vi "UHR-Fleezers Control (host) - 12.7d.vi"() -> ()   [LabVIEW 2012] (continued)
                                n2052 = case shown="True" w2961 {
                                tunnel: w2978 -> [_ w2993]
                                tunnel: w2977 -> [_ w2992]
                                tunnel: w2976 -> [_ w2982]
                                tunnel: w2975 -> [_ w2984]
                                frame False {
                                }
                                frame True {
                                n2053 = local read "Time (s)"() -> (w2983:dbl)
                                n2054 = case shown="\"Yank\"" w2992 {
                                tunnel: w2993 -> [_ w2996]
                                tunnel: w2984 -> [_ w2994]
                                frame "Image", Default {
                                }
                                frame "Yank" {
                                n2055 = flat-sequence {
                                tunnel: [w3002] -> w2997
                                tunnel: w2996 -> [w3002]
                                tunnel: [w2998] -> w2995
                                tunnel: w2994 -> [w2998]
                                tunnel: w2997 -> [w3005]
                                tunnel: w2995 -> [w3003]
                                frame #0 {
                                n2056 = local read "Yank Delay (s)"() -> (w3001:dbl)
                                n2057 = Multiply(x=w3001, y=1000.0) -> (x*y=w2999:dbl)
                                n2058 = Wait (ms)(milliseconds to wait=w2999) -> ()  [unwired: 1 out]
                                }
                                frame #1 {
                                n2059 = local read "Yank to which?"() -> (w3004:bool)
                                n2060 = case shown="False" w3004 {
                                tunnel: w3005 -> [_ w3032]
                                tunnel: w3003 -> [w3006 _]
                                frame False {
                                n2061 = flat-sequence {
                                tunnel: w3006 -> [w3007]
                                frame #0 {
                                n2062 = property on="Trap Pos FB SP" class="DigNum (strict)"("Val(Sgnl)"=w3007) -> ()  [unwired: 2 in, 2 out]
                                }
                                frame #1 {
                                n2063 = Wait (ms)(milliseconds to wait=u32 700) -> ()  [unwired: 1 out]
                                }
                                frame #2 {
                                n2064 = local read "Action (%)"() -> (w3012:dbl)
                                n2065 = Absolute Value(x=w3012) -> (abs(x)=w3011:dbl)
                                n2066 = Greater?(x=w3011, y=70.0) -> (0:w3009:bool)
                                n2067 = property on="Remove Action Offset" class="Bool (strict)"("Val(Sgnl)"=w3009) -> ()  [unwired: 2 in, 2 out]
                                }
                                frame #3 {
                                n2068 = for {
                                N: 4 -> [_]
                                n2069 = flat-sequence {
                                frame #0 {
                                n2070 = Wait (ms)(milliseconds to wait=u32 500) -> ()  [unwired: 1 out]
                                }
                                frame #1 {
                                n2071 = local read "Action (%)"() -> (w3018:dbl)
                                n2072 = Absolute Value(x=w3018) -> (abs(x)=w3017:dbl)
                                n2073 = Greater?(x=w3017, y=70.0) -> (0:w3015:bool)
                                n2074 = property on="Remove Action Offset" class="Bool (strict)"("Val(Sgnl)"=w3015) -> ()  [unwired: 2 in, 2 out]
                                }
                                }
                                }
                                }
                                frame #4 {
                                n2075 = local read "Shift confocal"() -> (w3023:bool)
                                n2076 = local read "Mean"() -> (w3025:dbl)
                                n2077 = Greater?(x=w3025, y=11.0) -> (0:w3022:bool)
                                n2078 = Not(x=w3022) -> (.not. x?=w3021:bool)
                                n2079 = And(x=w3022, y=w3023) -> (x .and. y?=w3020:bool)
                                n2080 = And(x=w3021, y=w3023) -> (x .and. y?=w3019:bool)
                                n2081 = case shown="True" w3020 {
                                frame False {
                                }
                                frame True {
                                n2082 = local read "Confocal Y 2 (V)"() -> (w3029:dbl)
                                n2083 = local read "Confocal X 2 (V)"() -> (w3028:dbl)
                                n2084 = property on="AO2" class="Slide (strict)"("Val(Sgnl)"=w3028) -> ()  [unwired: 2 in, 2 out]
                                n2085 = property on="AO1" class="Slide (strict)"("Val(Sgnl)"=w3029) -> ()  [unwired: 2 in, 2 out]
                                }
                                }
                                n2086 = case shown="True" w3019 {
                                frame False {
                                }
                                frame True {
                                n2087 = local read "Confocal X 1 (V)"() -> (w3026:dbl)
                                n2088 = local read "Confocal Y 1 (V)"() -> (w3027:dbl)
                                n2089 = property on="AO1" class="Slide (strict)"("Val(Sgnl)"=w3027) -> ()  [unwired: 2 in, 2 out]
                                n2090 = property on="AO2" class="Slide (strict)"("Val(Sgnl)"=w3026) -> ()  [unwired: 2 in, 2 out]
                                }
                                }
                                }
                                frame #5 {
                                n2091 = Wait (ms)(milliseconds to wait=u32 1500) -> ()  [unwired: 1 out]
                                }
                                frame #6 {
                                n2092 = property on="Rem fb disp offset" class="Bool (strict)"("Val(Sgnl)"=TRUE ("Value (Signaling)")) -> ()  [unwired: 2 in, 2 out]
                                }
                                }
                                }
                                frame True {
                                n2093 = flat-sequence {
                                tunnel: w3032 -> [w3033]
                                frame #0 {
                                n2094 = property on="Trap Delta (MHz)" class="DigNum (strict)"("Val(Sgnl)"=w3033) -> ()  [unwired: 2 in, 2 out]
                                }
                                frame #1 {
                                n2095 = Wait (ms)(milliseconds to wait=u32 500) -> ()  [unwired: 1 out]
                                }
                                frame #2 {
                                n2096 = local read "Shift confocal"() -> (w3039:bool)
                                n2097 = local read "Mean"() -> (w3041:dbl)
                                n2098 = Greater?(x=w3041, y=11.0) -> (0:w3038:bool)
                                n2099 = Not(x=w3038) -> (.not. x?=w3037:bool)
                                n2100 = And(x=w3038, y=w3039) -> (x .and. y?=w3036:bool)
                                n2101 = And(x=w3037, y=w3039) -> (x .and. y?=w3035:bool)
                                n2102 = case shown="True" w3036 {
                                frame False {
                                }
                                frame True {
                                n2103 = local read "Confocal Y 2 (V)"() -> (w3045:dbl)
                                n2104 = local read "Confocal X 2 (V)"() -> (w3044:dbl)
                                n2105 = property on="AO2" class="Slide (strict)"("Val(Sgnl)"=w3044) -> ()  [unwired: 2 in, 2 out]
                                n2106 = property on="AO1" class="Slide (strict)"("Val(Sgnl)"=w3045) -> ()  [unwired: 2 in, 2 out]
                                }
                                }
                                n2107 = case shown="True" w3035 {
                                frame False {
                                }
                                frame True {
                                n2108 = local read "Confocal Y 1 (V)"() -> (w3043:dbl)
                                n2109 = local read "Confocal X 1 (V)"() -> (w3042:dbl)
                                n2110 = property on="AO2" class="Slide (strict)"("Val(Sgnl)"=w3042) -> ()  [unwired: 2 in, 2 out]
                                n2111 = property on="AO1" class="Slide (strict)"("Val(Sgnl)"=w3043) -> ()  [unwired: 2 in, 2 out]
                                }
                                }
                                }
                                }
                                }
                                }
                                }
                                }
                                }
                                }
                                n2112 = local read "Messages"() -> (w2991:string)
                                n2113 = Subtract(x=w2983, y=w2982) -> (x-y=w2989:dbl)
                                "Duration (s)" <- w2989
                                n2114 = Number To Decimal String(number=w2989, width (-)=i16 0) -> (decimal integer string=w2987:string)
                                n2115 = Concatenate Strings(w2987, " s fluorescence event." ("string")) -> (w2985:string)
                                n2116 = call "Update messages.vi"("Message to add"=w2985, "Old message string"=w2991) -> ("New message string"=w2990:string)
                                n2117 = local write "Reset Force"(FALSE ("Reset Force")) -> ()
                                n2118 = local write "Waiting"(TRUE ("Waiting")) -> ()
                                n2119 = local write "Messages"(w2990) -> ()
                                n2120 = local write "Fl. High"(FALSE ("Fl. High")) -> ()
                                n2121 = call <vilib>:"Beep.vi"() -> ()  [unwired: 3 in, 9 out]
                                }
                                }
                                n2122 = node-c288() -> ()  [unwired: 2 out]
                              }
                              n2123 = node-c288(w2959) -> ()  [unwired: 1 out]
                            }
                          }
                        }
                      }
                      n2124 = local read "Trap Delta (MHz)"() -> (w2874:dbl)
                      n2125 = local read "Trap Pos FB SP"() -> (w2869:fxp<+/-,16,1>)
                    }
                  }
                }
                frame #1 {
                  n2126 = local read "Stop All"() -> (w3055:bool)
                  n2127 = local read "Fl. Triggered..."() -> (w3053:bool)
                  n2128 = Not(x=w3053) -> (.not. x?=w3054:bool)
                  n2129 = Or(x=w3054, y=w3055) -> (x .or. y?=w3052:bool)
                }
              }
              n2130 = case shown="True" w2646 {
                frame False {
                }
                frame True {
                  n2131 = local read "Confocal Y 1 (V)"() -> (w2656:dbl)
                  n2132 = local read "Confocal X 1 (V)"() -> (w2655:dbl)
                  n2133 = property on="AO2" class="Slide (strict)"("Val(Sgnl)"=w2655) -> ()  [unwired: 2 in, 2 out]
                  n2134 = property on="AO1" class="Slide (strict)"("Val(Sgnl)"=w2656) -> ()  [unwired: 2 in, 2 out]
                }
              }
              n2135 = case shown="True" w2646 {
                frame False {
                }
                frame True {
                  w2654 = FALSE ("Fl. High")
                  n2136 = local write "Waiting"(w2654) -> ()
                  n2137 = local write "Fl. High"(w2654) -> ()
                }
              }
              n2138 = node-c288() -> ()  [unwired: 2 out]
            }
            n2139 = node-c288(w2644) -> ()  [unwired: 1 out]
          }
        }
      }
      event "Stop All": Value Change {
        n2140 = event-data() -> ()  [unwired: 7 out]
        n2141 = local read "Stop All"() -> (w3060:bool)
      }
    }
    n2142 = node-c288() -> ()  [unwired: 2 out]
  }
  n2143 = timed-loop "Mouse control: trap position (AOM deflection), set confocal spot from image" {
    tunnel: [w3062] -> w74
    timing: w68 -> [_]
    timing-out: [_] -> w67
    tunnel: w5 -> [w3061]
    stop <- w3062 stop-if-true
    n2144 = node-c288() -> ()  [unwired: 2 out]
    n2145 = event shown="[0] \"Pane\": Mouse Down" {
      selector: _ -> [_ _]
      dyn-events: _ -> [_ _]
      timeout: _ -> [_ _]
      tunnel: w3061 -> [w3065 _]
      event Mouse Down {
        n2146 = event-data() -> ("Time"=w3067:u32, "Coords"=w3066:T7, "Button"=w3068:u16)  [unwired: 6 out]
        n2147 = case shown="3" w3068 {
          tunnel: w3067 -> [_ _ w3174]
          tunnel: w3066 -> [_ w3105 w3172]
          tunnel: w3065 -> [_ _ w3168]
          frame 0, Default {
          }
          frame 1 {
            n2148 = property on="APD 2" class="ImageControl"() -> ("Displayed Image Position"=w3075:cluster{"Left":i32, "Top":i32})  [unwired: 2 in, 2 out]
            n2149 = property on="APD 1" class="ImageControl"() -> ("Displayed Image Position"=w3104:cluster{"Left":i32, "Top":i32})  [unwired: 2 in, 2 out]
            n2150 = property on="Detection Laser X" class="ImageControl"() -> ("Displayed Image Position"=w3101:cluster{"Left":i32, "Top":i32})  [unwired: 2 in, 2 out]
            n2151 = property on="Detection Laser Y" class="ImageControl"() -> ("Displayed Image Position"=w3100:cluster{"Left":i32, "Top":i32})  [unwired: 2 in, 2 out]
            n2152 = property on="APD 2" class="ImageControl"() -> ("Displayed Image Size"=w3074:cluster{"Width":u32, "Height":u32})  [unwired: 2 in, 2 out]
            n2153 = property on="APD 1" class="ImageControl"() -> ("Displayed Image Size"=w3102:cluster{"Width":u32, "Height":u32})  [unwired: 2 in, 2 out]
            n2154 = property on="Detection Laser X" class="ImageControl"() -> ("Displayed Image Size"=w3103:cluster{"Width":u32, "Height":u32})  [unwired: 2 in, 2 out]
            n2155 = property on="Detection Laser Y" class="ImageControl"() -> ("Displayed Image Size"=w3099:cluster{"Width":u32, "Height":u32})  [unwired: 2 in, 2 out]
            n2156 = Unbundle By Name(w3074) -> ("Width"=w3071:u32, "Height"=w3070:u32)
            n2157 = Unbundle By Name(w3075) -> ("Left"=w3073:i32, "Top"=w3072:i32)
            n2158 = Unbundle By Name(w3102) -> ("Width"=w3096:u32, "Height"=w3095:u32)
            n2159 = Unbundle By Name(w3103) -> ("Width"=w3092:u32, "Height"=w3091:u32)
            n2160 = Unbundle By Name(w3099) -> ("Width"=w3088:u32, "Height"=w3087:u32)
            n2161 = Unbundle By Name(w3104) -> ("Left"=w3098:i32, "Top"=w3097:i32)
            n2162 = Unbundle By Name(w3101) -> ("Left"=w3094:i32, "Top"=w3093:i32)
            n2163 = Unbundle By Name(w3100) -> ("Left"=w3090:i32, "Top"=w3089:i32)
            n2164 = Bundle("Left"=w3073, "Top"=w3072, "Width"=w3071, "Height"=w3070) -> (w3069:T33)  [unwired: 1 in]
            n2165 = Bundle("Left"=w3098, "Top"=w3097, "Width"=w3096, "Height"=w3095) -> (w3086:T33)  [unwired: 1 in]
            n2166 = Bundle("Left"=w3094, "Top"=w3093, "Width"=w3092, "Height"=w3091) -> (w3085:T33)  [unwired: 1 in]
            n2167 = Bundle("Left"=w3090, "Top"=w3089, "Width"=w3088, "Height"=w3087) -> (w3084:T33)  [unwired: 1 in]
            n2168 = Build Cluster Array(w3069, w3086, w3085, w3084) -> (w3083:T34)
            n2169 = for {
              tunnel: w3105 -> [w3116]
              tunnel: w3083 -> [w3117] mode=indexing
              shift-right: [w3114] -> w3081
              shift-left: TRUE -> [w3115]
              shift-right: [w3113] -> w3079
              shift-left: _ -> [w3109]
              shift-right: [w3112] -> w3078
              shift-left: _ -> [w3108]
              shift-right: [w3111] -> w3077
              shift-left: _ -> [w3107]
              shift-right: [w3110] -> w3076
              shift-left: _ -> [w3106]
              n2170 = case shown="True" w3115 {
                selector: w3115 -> [w3122 _]
                tunnel: w3117 -> [_ w3131]
                tunnel: w3116 -> [_ w3129]
                tunnel: [w3122 w3127] -> w3114
                tunnel: [w3121 w3126] -> w3113
                tunnel: [w3120 w3125] -> w3112
                tunnel: [w3119 w3124] -> w3111
                tunnel: [w3118 w3123] -> w3110
                tunnel: w3109 -> [w3121 _]
                tunnel: w3108 -> [w3120 _]
                tunnel: w3107 -> [w3119 _]
                tunnel: w3106 -> [w3118 _]
                frame False {
                }
                frame True {
                  n2171 = Unbundle(w3131) -> (w3130:T33)
                  n2172 = call "isclickinwindow.vi"("Image Param"=w3130, "Point32"=w3129) -> ("4 Y"=w3123:i32, "3 Height"=w3124:i32, "2 X"=w3125:i32, "1 Width"=w3126:i32, "In image?"=w3128:bool)  [unwired: 1 in]
                  n2173 = Not(x=w3128) -> (.not. x?=w3127:bool)
                }
              }
            }
            n2174 = Not(x=w3081) -> (.not. x?=w3080:bool)
            n2175 = case shown="True" w3080 {
              tunnel: w3078 -> [_ w3145]
              tunnel: w3076 -> [_ w3144]
              tunnel: w3079 -> [_ w3143]
              tunnel: w3077 -> [_ w3142]
              frame False {
              }
              frame True {
                w3132 = FALSE ("Get Point")
                n2176 = local read "Scan lines (y)"() -> (w3147:u64)
                n2177 = disable-structure shown="Disabled" {
                  frame Disabled {
                  }
                  frame Enabled {
                  }
                }
                n2178 = local read "Actual MCL Inc (V)"() -> (w3141:dbl)
                n2179 = local read "Scan steps (MCL)"() -> (w3146:u64)
                n2180 = Divide "Y Pix/step"(x=w3142, y=w3147) -> (x/y=w3154:dbl)
                n2181 = Divide "Y V/pix"(x=w3141, y=w3154) -> (x/y=w3153:dbl)
                n2182 = Divide "Y half step offset"(x=w3141, y=2.0) -> (x/y=w3155:dbl)
                n2183 = Divide "X pix/step"(x=w3143, y=w3146) -> (x/y=w3152:dbl)
                n2184 = Negate(x=w3155) -> (-x=w3156:dbl)
                n2185 = local read "Initial Y"() -> (w3162:dbl)
                n2186 = Multiply(x=w3144, y=w3153) -> (x*y=w3163:dbl)
                n2187 = Divide "X half step offset"(x=w3141, y=2.0) -> (x/y=w3149:dbl)
                n2188 = Divide "X V/pix"(x=w3141, y=w3152) -> (x/y=w3151:dbl)
                n2189 = Multiply(x=w3141, y=w3146) -> (x*y=w3158:dbl)
                n2190 = Compound Arithmetic op=ADD(w3156, w3163, w3162) -> (w3133:dbl)
                "Pointer Y (V)" <- w3133
                n2191 = Multiply(x=w3151, y=w3145) -> (x*y=w3160:dbl)
                n2192 = Negate(x=w3149) -> (-x=w3148:dbl)
                n2193 = local read "Initial X"() -> (w3161:dbl)
                n2194 = Negate(x=w3160) -> (-x=w3159:dbl)
                n2195 = Compound Arithmetic op=ADD(w3148, w3158, w3161, w3159) -> (w3134:dbl)
                "Pointer X (V)" <- w3134
                n2196 = case shown="True" "Set High F Confocal Spot (X-Y)" {
                  tunnel: w3134 -> [_ w3164]
                  tunnel: w3133 -> [_ w3165]
                  frame False {
                  }
                  frame True {
                    "Confocal Y 2 (V)" <- w3165
                    "Confocal X 2 (V)" <- w3164
                  }
                }
                n2197 = Or(x="Set X Only", y="Set Confocal Spot (X-Y)") -> (x .or. y?=w3137:bool)
                n2198 = Or(x="Set Confocal Spot (X-Y)", y="Set Y Only") -> (x .or. y?=w3136:bool)
                n2199 = case shown="True" w3137 {
                  tunnel: w3134 -> [_ w3166]
                  frame False {
                  }
                  frame True {
                    n2200 = property on="AO2" class="Slide (strict)"("Val(Sgnl)"=w3166) -> ()  [unwired: 2 in, 2 out]
                    "Confocal X 1 (V)" <- w3166
                  }
                }
                n2201 = case shown="True" w3136 {
                  tunnel: w3133 -> [_ w3167]
                  frame False {
                  }
                  frame True {
                    n2202 = property on="AO1" class="Slide (strict)"("Val(Sgnl)"=w3167) -> ()  [unwired: 2 in, 2 out]
                    "Confocal Y 1 (V)" <- w3167
                  }
                }
                n2203 = local write "Set High F Confocal Spot (X-Y)"(w3132) -> ()
                n2204 = local write "Set Confocal Spot (X-Y)"(w3132) -> ()
                n2205 = local write "Set X Only"(w3132) -> ()
                n2206 = local write "Set Y Only"(w3132) -> ()
              }
            }
          }
          frame 3 {
            n2207 = local read "BD 2 Frequency 1 (MHz)"() -> (w3169:dbl)
            n2208 = local read "BD 1 Frequency 1 (MHz)"() -> (w3170:dbl)
            n2209 = local write "Manipulating Trap"(TRUE ("Manipulating Trap")) -> ()
            n2210 = local write "Coords"(T7 {"Horizontal"=0, "Vertical"=0} ("Coords")) -> ()
            n2211 = while {
              tunnel: w3174 -> [w3179]
              tunnel: w3172 -> [w3178]
              tunnel: w3170 -> [w3177]
              tunnel: w3169 -> [w3176]
              tunnel: w3168 -> [w3175]
              stop <- w3180 stop-if-true
              n2212 = event shown="[0] \"Pane\": Mouse Move" {
                selector: _ -> [_ _]
                dyn-events: _ -> [_ _]
                timeout: _ -> [_ _]
                tunnel: ["Force Manip Abort" w3244] -> w3180
                tunnel: w3179 -> [w3187 _]
                tunnel: w3178 -> [w3185 _]
                tunnel: w3177 -> [w3184 _]
                tunnel: w3176 -> [w3183 _]
                tunnel: w3175 -> [w3181 _]
                event Mouse Move {
                  n2213 = event-data() -> ("Time"=w3188:u32, "Coords"=w3189:T7)  [unwired: 3 out]
                  n2214 = Less?(x=w3188, y=w3187) -> (x < y?=w3186:bool)
                  n2215 = case "Makes sure old motion events prior to mouse click aren't used" shown="False" w3186 {
                    tunnel: w3189 -> [w3231 _]
                    tunnel: w3185 -> [w3232 _]
                    tunnel: w3184 -> [w3206 _]
                    tunnel: w3183 -> [w3205 _]
                    tunnel: w3181 -> [w3190 _]
                    frame False {
                      n2216 = Subtract(x=w3231, y=w3232) -> (x-y=w3230:T7)
                      "Coords" <- w3230
                      n2217 = local read "Y RF Frequency Limits (MHz)"() -> (w3191:T16)
                      n2218 = To Double Precision Float(number=w3230) -> (double precision float=w3229:cluster{"Horizontal":dbl, "Vertical":dbl})
                      n2219 = Multiply(x=cluster{"Horizontal":dbl, "Vertical":dbl} {"Horizontal"=-1.0, "Vertical"=1.0}, y="Manipulation Scaling") -> (x*y=w3225:cluster{"Horizontal":dbl, "Vertical":dbl})
                      n2220 = local read "X RF Frequency Limits (MHz)"() -> (w3192:T16)
                      n2221 = Multiply(x=w3229, y=w3225) -> (x*y=w3227:cluster{"Horizontal":dbl, "Vertical":dbl})
                      n2222 = Unbundle By Name(w3227) -> ("Horizontal"=w3222:dbl, "Vertical"=w3226:dbl)
                      n2223 = Unbundle By Name(w3191) -> ("Maximum"=w3194:dbl, "Minimum"=w3193:dbl)
                      n2224 = Boolean To (0,1)(Boolean="Manip. X?") -> (0, 1=w3220:i16)
                      n2225 = Boolean To (0,1)(Boolean="Manip. Y?") -> (0, 1=w3217:i16)
                      n2226 = local read "BD 1 Frequency 2 (MHz)"() -> (w3208:dbl)
                      n2227 = Multiply(x=w3226, y=w3217) -> (x*y=w3219:dbl)
                      n2228 = Multiply(x=w3220, y=w3222) -> (x*y=w3223:dbl)
                      n2229 = local read "BD 2 Frequency 2 (MHz)"() -> (w3207:dbl)
                      n2230 = Unbundle By Name(w3192) -> ("Maximum"=w3196:dbl, "Minimum"=w3195:dbl)
                      n2231 = Add(x=w3205, y=w3219) -> (x+y=w3198:dbl)
                      n2232 = Add(x=w3206, y=w3223) -> (x+y=w3200:dbl)
                      n2233 = In Range and Coerce(upper limit=w3196, x=w3200, lower limit=w3195) -> (coerced(x)=w3199:dbl)  [unwired: 1 out]
                      n2234 = In Range and Coerce(upper limit=w3194, x=w3198, lower limit=w3193) -> (coerced(x)=w3197:dbl)  [unwired: 1 out]
                      n2235 = Subtract(x=w3199, y=w3208) -> (x-y=w3216:dbl)
                      n2236 = Subtract(x=w3197, y=w3207) -> (x-y=w3215:dbl)
                      n2237 = Square(x=w3216) -> (x^2=w3214:dbl)
                      n2238 = Square(x=w3215) -> (x^2=w3213:dbl)
                      n2239 = Add(x=w3214, y=w3213) -> (x+y=w3212:dbl)
                      n2240 = Square Root(x=w3212) -> (sqrt(x)=w3209:dbl)
                      n2241 = In Range and Coerce(upper limit="Limit Max (MHz)", x=w3209, lower limit="Limit Min (MHz)") -> (In Range?=w3202:bool)  [unwired: 1 out]
                      n2242 = Not(x="Limits Enable") -> (.not. x?=w3201:bool)
                      n2243 = Or(x=w3202, y=w3201) -> (x .or. y?=w3203:bool)
                      n2244 = case shown="True" w3203 {
                        tunnel: w3209 -> [_ w3234]
                        tunnel: w3199 -> [_ w3241]
                        tunnel: w3208 -> [_ w3240]
                        tunnel: w3197 -> [_ w3239]
                        tunnel: w3207 -> [_ w3238]
                        tunnel: w3192 -> [_ w3236]
                        tunnel: w3191 -> [_ w3235]
                        tunnel: w3190 -> [_ w3233]
                        frame False {
                        }
                        frame True {
                          n2245 = local read "BD 1 Frequency 3 (MHz)"() -> (w3242:dbl)
                          n2246 = local read "BD 2 Frequency 3 (MHz)"() -> (w3237:dbl)
                          n2247 = local write "Trap Delta (MHz)"(w3234) -> ()
                          n2248 = call "set RF board frequency - interlace.vi"("Board 2 Frequency Limits"=w3235, "Board 1 Frequency Limits"=w3236, "FPGA VI Reference In"=w3233, "Board 2 Frequency 3 (MHz)"=w3237, "Board 1 Frequency 3 (MHz)"=w3242, "Board 2 Frequency 2 (MHz)"=w3238, "Board 2 Frequency 1 (MHz)"=w3239, "Board 1 Frequency 2 (MHz)"=w3240, "Board 1 Frequency 1  (MHz)"=w3241) -> ()  [unwired: 1 in, 2 out]
                          n2249 = local write "BD 2 Frequency 1 (MHz)"(w3239) -> ()
                          n2250 = local write "BD 1 Frequency 1 (MHz)"(w3241) -> ()
                        }
                      }
                    }
                    frame True {
                    }
                  }
                }
                event Mouse Up {
                  n2251 = event-data() -> ("Button"=w3243:u16)  [unwired: 8 out]
                  n2252 = case shown="3" w3243 {
                    tunnel: [FALSE TRUE] -> w3244
                    frame 0, Default {
                    }
                    frame 3 {
                      n2253 = local read "Trap Delta (MHz)"() -> (w3246:dbl)
                      n2254 = property on="Initial delta (MHz)" class="DigNum (strict)"("Val(Sgnl)"=w3246) -> ()  [unwired: 2 in, 2 out]
                      n2255 = local write "Manipulating Trap"(FALSE ("Manipulating Trap")) -> ()
                    }
                  }
                }
              }
            }
          }
        }
      }
      event Mouse Move {
        n2256 = event-data() -> ()  [unwired: 6 out]
      }
    }
    n2257 = local read "Stop All"() -> (w3062:bool)
    n2258 = node-c288() -> ()  [unwired: 2 out]
  }
  n2259 = flat-sequence "Video" {
    tunnel: [w3258] -> w55
    tunnel: w55 -> [w3298]
    frame #0 {
      n2260 = while {
        stop <- w3250 continue-if-true
        n2261 = call "Close Video Capture.vi"() -> ("error code OUT"=w3252:i32)
        n2262 = Equal?(x=w3252, y=0) -> (x = y?=w3250:bool)
      }
      n2263 = local write "Stop All"(FALSE ("Stop All")) -> ()
    }
    frame #1 {
      n2264 = call "DMR_Init.vi"() -> ()  [unwired: 3 out]
    }
    frame #2 {
      w3253 = "DE245428202"  # MSU fleezers card #
      (unwired) "DE019116701"  # Illinois fleezers card #
      # "Setting the destination format to Mono8 makes sure that the image can be displayed in the intensity plot."
      n2265 = call "DMR_GetDevice.vi"("search string IN"=w3253) -> ("device handle OUT"=w3276:i32)  [unwired: 4 in, 2 out]
      n2266 = call "DMR_OpenDevice.vi"("device handle IN"=w3276) -> ("driver handle OUT"=w3259:i32)  [unwired: 4 out]
      n2267 = call "DMR_FindList.vi"("flags IN"=u32 0 ("flags"), "list name IN"="" ("String"), "list type IN"=T35."camera descriptions", "driver handle IN"=w3259) -> ("list handle OUT"=w3262:i32)  [unwired: 2 out]
      n2268 = call "DMR_FindList.vi"("flags IN"=u32 0 ("flags"), "list name IN"="Base", "list type IN"=T35."setting", "driver handle IN"=w3259) -> ("list handle OUT"=w3260:i32)  [unwired: 2 out]
      n2269 = call "OBJ_GetHandle.vi"("object name IN"="VideoStandard", "list handle IN"=w3262) -> ("object handle OUT"=w3256:i32)  [unwired: 3 out]
      n2270 = call "OBJ_GetHandle.vi"("object name IN"="PixelFormat", "list handle IN"=w3260) -> ("object handle OUT"=w3270:i32)  [unwired: 3 out]
      n2271 = call "OBJ_SetS.vi"("value index IN"=0, "value IN"="NTSC M", "object handle IN"=w3256) -> ()  [unwired: 2 out]
      n2272 = call "OBJ_SetS.vi"("value index IN"=0, "value IN"="Mono8" ("value"), "object handle IN"=w3270) -> ()  [unwired: 2 out]
      n2273 = call "OBJ_GetHandle.vi"("object name IN"="VideoChannel", "list handle IN"=w3260) -> ("object handle OUT"=w3266:i32)  [unwired: 3 out]
      n2274 = while {
        tunnel: [w3280] -> w3258
        tunnel: w3259 -> [w3277]
        stop <- w3278 continue-if-true
        n2275 = call "DMR_ImageRequestSingle.vi"("request control IN"=0, "driver handle IN"=w3277) -> ("error code OUT"=w3279:i32, "driver handle OUT"=w3280:i32)  [unwired: 2 out]
        n2276 = Equal To 0?(x=w3279) -> (x = 0?=w3278:bool)
      }
      n2277 = call "OBJ_SetI.vi"("value index IN"=0, "value IN"=3 ("Video channel"), "object handle IN"=w3266) -> ()  [unwired: 2 out]
    }
    frame #3 {
      w3286 = T19 0 items=["Grayscale (U8)", "Grayscale (I16)", "Grayscale (SGL)", "Complex (CSG)", "RGB (U32)", "HSL (U32)", "RGB (U64)"] ("Image Type")
      w3294 = T19 0 items=["Grayscale (U8)", "Grayscale (I16)", "Grayscale (SGL)", "Complex (CSG)", "RGB (U32)", "HSL (U32)", "RGB (U64)"] ("Image Type")
      n2278 = for "Create Greyscale map" {
        N: 256 -> [_]
        tunnel: [w3300] -> w3283 mode=indexing
        workers-P: _ -> [_]
        i -> [w3303]
        n2279 = To Unsigned Byte Integer(number=w3303) -> (unsigned 8bit integer=w3299:u8)
        n2280 = Join Numbers(hi=w3299, lo=w3299) -> ((hi.lo)=w3302:u16)
        n2281 = Join Numbers(hi=w3299, lo=w3299) -> ((hi.lo)=w3301:u16)
        n2282 = Join Numbers(hi=w3302, lo=w3301) -> ((hi.lo)=w3300:u32)
      }
      n2283 = call "IMAQ Create"("Image Name"="Scaled video", "Image Type"=w3286) -> ("New Image"=w3285:T2)  [unwired: 2 in, 2 out]
      n2284 = call "IMAQ Create"("Image Name"="Main video", "Image Type"=w3294) -> ("New Image"=w3295:T2)  [unwired: 2 in, 2 out]
      n2285 = node-c288(0 ("Processor")) -> (w3293:T23)  [unwired: 3 out]
      n2286 = Initialize Array(u32 0 ("Window Number (0...15)"), 480 ("dimension size"), 640 ("dimension size")) -> (w3288:u32[][])
      n2287 = timed-loop {
        tunnel: w3298 -> [w3320]
        tunnel: [w3319] -> w3297
        tunnel: w3295 -> [w3318]
        timing: w3293 -> [_]
        timing-out: [_] -> w3292
        tunnel: w3288 -> [w3307]
        tunnel: w3285 -> [w3305]
        tunnel: w3283 -> [w3304]
        stop <- w3306 stop-if-true
        # "This block performs the \nactual image capture."
        n2288 = node-c288() -> ()  [unwired: 2 out]
        n2289 = local read "Stop All"() -> (w3306:bool)
        n2290 = Reciprocal(x="Video Capture Rate (Hz)") -> (1/x=w3310:dbl)
        n2291 = Multiply(x=w3310, y=1000.0) -> (x*y=w3308:dbl)
        n2292 = call "DMR_ImageRequestWaitFor.vi"("queue number IN"=0, "timeout(ms) IN"=500, "driver handle IN"=w3320) -> ("error code OUT"=w3324:i32, "request number OUT"=w3321:i32, "driver handle OUT"=w3322:i32)
        n2293 = feedback #1(T36 refnum ("Avi Refnum")) -> (w3312:T36)
        n2294 = case shown="True" "New Video File" {
          tunnel: [T36 refnum ("Avi Refnum") w3341] -> w3314
          tunnel: [FALSE TRUE] -> w3315
          tunnel: w3312 -> [_ w3337]
          frame False {
          }
          frame True {
            n2295 = call "Create new save file.vi"("Ext"=".avi" ("string"), "Index In"="Video Index") -> ("Path Out"=w3333:path, "Index Out"=w3334:dbl)  [unwired: 1 in]
            "Path Out" <- w3333
            n2296 = Not Equal?(x=w3337, y=T36 refnum ("Avi Refnum")) -> (x != y?=w3338:bool)
            n2297 = Increment(x=w3334) -> (x+1=w3343:dbl)
            n2298 = case shown="True" w3338 {
              tunnel: w3337 -> [_ w3344]
              frame False {
              }
              frame True {
                n2299 = call "IMAQ AVI Close"("Avi Refnum"=w3344) -> ()  [unwired: 1 in, 10 out]
              }
            }
            n2300 = local write "Video Index"(w3343) -> ()
            n2301 = call "IMAQ AVI Create"("Frames Per Second"=u32 30, "AVI Path"=w3333) -> ("Avi Refnum"=w3341:T36)  [unwired: 5 in, 4 out]
          }
        }
        n2302 = Equal To 0?(x=w3324) -> (x = 0?=w3323:bool)
        n2303 = Select(t=w3314, s=w3315, f=w3312) -> (s? t:f=w3313:T36)
        n2304 = feedback-in #1(w3313) -> ()
        n2305 = case shown="True" w3323 {
          tunnel: w3322 -> [w3345 w3379]
          tunnel: w3321 -> [_ w3378]
          tunnel: [w3345 w3375] -> w3319
          tunnel: w3318 -> [_ w3360]
          tunnel: w3307 -> [_ w3364]
          tunnel: w3313 -> [_ w3362]
          tunnel: w3305 -> [_ w3357]
          tunnel: w3304 -> [_ w3356]
          frame False {
          }
          frame True {
            w3369 = u32 0 ("X-offset IN")
            n2306 = call "DMR_GetImageRequestBufferData.vi"("driver handle IN"=w3379, "request number IN"=w3378) -> ("width OUT"=w3368:i32, "height OUT"=w3367:i32, "driver handle OUT"=w3374:i32, "request number OUT"=w3373:i32, "bytes per pixel OUT"=w3370:i32)  [unwired: 13 out]
            n2307 = call "DMR_GetImageRequestBufferImageData.vi"("driver handle IN"=w3374, "request number IN"=w3373, "bytes per pixel IN"=w3370, "X-offset IN"=w3369, "Y-offset IN"=w3369, "height IN"=w3367, "width IN"=w3368) -> ("driver handle OUT"=w3372:u32, "request number OUT"=w3371:u32, "image OUT"=w3349:u32[][])  [unwired: 10 out]
            n2308 = Transpose 2D Array(2D array=w3349) -> (transposed array=w3355:u32[][])
            n2309 = Select(t=w3355, s="Flip Y (or X)", f=w3349) -> (s? t:f=w3354:u32[][])
            n2310 = call "DMR_ImageRequestUnlock.vi"("request number IN"=w3371, "driver handle IN"=w3372) -> ("driver handle OUT"=w3377:i32)  [unwired: 1 in, 2 out]
            n2311 = for {
              tunnel: w3354 -> [w3414] mode=indexing
              tunnel: [w3413] -> w3352 mode=indexing
              n2312 = Reverse 1D Array(array=w3414) -> (reversed array=w3413:u32[])
            }
            n2313 = call "DMR_ImageRequestSingle.vi"("request control IN"=0, "driver handle IN"=w3377) -> ("driver handle OUT"=w3375:i32)  [unwired: 3 out]
            n2314 = Transpose 2D Array(2D array=w3352) -> (transposed array=w3353:u32[][])
            n2315 = Select(t=w3353, s="Flip Y (or X)", f=w3352) -> (s? t:f=w3350:u32[][])
            n2316 = Select(t=w3350, s="Flip Image", f=w3349) -> (s? t:f=w3347:u32[][])
            n2317 = case shown="True" "Averaging" {
              tunnel: w3347 -> [w3417 w3422]
              tunnel: [w3417 w3421] -> w3361
              tunnel: w3364 -> [_ w3419]
              frame False {
              }
              frame True {
                (unwired) 1
                w3427 = 1
                n2318 = feedback #2(w3419) -> (w3418:u32[][])
                n2319 = Add(x=w3422, y=w3418) -> (x+y=w3423:u32[][])
                n2320 = Select(t=w3419, s="Reset Averaging", f=w3423) -> (s? t:f=w3425:u32[][])
                n2321 = feedback-in #2(w3425) -> ()
                n2322 = feedback #3(w3427) -> (w3420:i32)
                n2323 = Divide(x=w3423, y=w3420) -> (x/y=w3424:dbl[][])
                n2324 = Increment(x=w3420) -> (x+1=w3428:i32)
                n2325 = To Unsigned Long Integer(number=w3424) -> (unsigned 32bit integer=w3421:u32[][])
                n2326 = Select(t=w3427, s="Reset Averaging", f=w3428) -> (s? t:f=w3426:i32)
                n2327 = feedback-in #3(w3426) -> ()
              }
            }
            n2328 = case shown="True" "Zoom video window" {
              tunnel: w3361 -> [_ w3393]
              tunnel: w3357 -> [_ w3392]
              frame False {
              }
              frame True {
                n2329 = To Double Precision Float(number=w3393) -> (double precision float=w3390:dbl[][])
                n2330 = In Range and Coerce(upper limit="Intensity Upper", x=w3390, lower limit="Intensity Lower") -> (coerced(x)=w3389:dbl[][])  [unwired: 1 out]
                n2331 = Subtract(x="Intensity Upper", y="Intensity Lower") -> (x-y=w3386:dbl)
                n2332 = Subtract(x=w3389, y="Intensity Lower") -> (x-y=w3387:dbl[][])
                n2333 = Divide(x=w3387, y=w3386) -> (x/y=w3388:dbl[][])
                n2334 = Multiply(x=255.0, y=w3388) -> (x*y=w3384:dbl[][])
                n2335 = To Unsigned Byte Integer(number=w3384) -> (unsigned 8bit integer=w3391:u8[][])
                n2336 = call "IMAQ ArrayToImage"("Image Pixels (U8)"=w3391, "Image"=w3392) -> ("Image Out"=w3380:T2)  [unwired: 4 in, 5 out]
                n2337 = First Call?() -> (First Call?: T/F=w3381:bool)
                n2338 = case shown="True" w3381 {
                  tunnel: w3380 -> [w3394 w3405]
                  frame False {
                    n2339 = flat-sequence {
                      tunnel: w3394 -> [w3400]
                      frame #0 {
                        w3397 = FALSE ("Get/Set Status? (Set)")
                        w3396 = 0 ("Window Number (0...15)")
                        n2340 = call "IMAQ WindSize"("Get/Set Status? (Set)"=w3397, "Window Number"=w3396) -> ("Width & Height out"=→"Window Size":cluster{"Width":i32, "Height":i32})  [unwired: 4 in, 2 out]
                        n2341 = call "IMAQ WindMove"("Window Number (0...15)"=w3396, "Get/Set Status? (Set)"=w3397) -> ("Coordinates (screen)"=→"Window Position":cluster{"X Position":i32, "Y Position":i32})  [unwired: 3 in, 1 out]
                        n2342 = call "IMAQ WindDraw"("Resize to Image Size? (Y)"=FALSE, "Window Number (0...15)"=w3396, "Image"=w3400) -> ()  [unwired: 7 in, 2 out]
                      }
                      frame #1 {
                        n2343 = call "IMAQ WindZoom 2"("Center Point"="Center Point", "Zoom to Fit? (False)"=FALSE, "Zoom Factor"="Zoom Factor") -> ()  [unwired: 5 in, 4 out]
                      }
                    }
                  }
                  frame True {
                    n2344 = flat-sequence {
                      tunnel: w3405 -> [w3408]
                      tunnel: [w3406] -> w3404
                      tunnel: w3404 -> [w3410]
                      frame #0 {
                        w3407 = TRUE ("Resize to Image Size? (Y)")
                        w3406 = 0 ("Window Number (0...15)")
                        n2345 = call "IMAQ WindNonTearing"("Window Number"=w3406, "NonTearing? (True)"=w3407) -> ()  [unwired: 8 in, 2 out]
                        n2346 = call "IMAQ WindDraw"("Resize to Image Size? (Y)"=w3407, "Window Number (0...15)"=w3406, "Image"=w3408) -> ()  [unwired: 7 in, 2 out]
                      }
                      frame #1 {
                        n2347 = call "IMAQ WindSize"("Scrollbars? (N)"=FALSE, "Width & Height"="Initial Window Size", "Window Number"=w3410) -> ()  [unwired: 3 in, 3 out]
                        n2348 = call "IMAQ WindMove"("Window Number (0...15)"=w3410, "Coordinates (screen)"="Initial Window Position") -> ()  [unwired: 3 in, 2 out]
                      }
                    }
                  }
                }
              }
            }
            n2349 = To Unsigned Byte Integer(number=w3361) -> (unsigned 8bit integer=w3359:u8[][])
            n2350 = call "IMAQ ArrayToImage"("Image Pixels (U8)"=w3359, "Image"=w3360) -> ("Image Out"=w3358:T2)  [unwired: 4 in, 5 out]
            "Primary Video Display" <- w3358
            n2351 = case shown="True" "Save Video" {
              tunnel: w3362 -> [_ w3416]
              tunnel: w3358 -> [_ w3415]
              frame False {
              }
              frame True {
                n2352 = call "IMAQ AVI Write Frame"("Image"=w3415, "Avi Refnum"=w3416) -> ()  [unwired: 2 in, 8 out]
              }
            }
            n2353 = case shown="True" "Save Image" {
              tunnel: w3359 -> [_ w3431]
              tunnel: w3356 -> [_ w3430]
              frame False {
              }
              frame True {
                n2354 = call <vilib>:"Flatten Pixmap.vi"("colors"=w3430, "8-bit pixmap"=w3431) -> ("image data"=w3437:T37)  [unwired: 4 in, 5 out]
                n2355 = call "Create new save file.vi"("Insert"="video_frame_" ("string"), "Ext"=".bmp" ("string"), "Index In"="Image Index") -> ("Path Out"=w3433:path, "Index Out"=w3438:dbl)
                n2356 = Increment(x=w3438) -> (x+1=w3432:dbl)
                n2357 = local write "Image Index"(w3432) -> ()
                n2358 = call <vilib>:"Write BMP File.vi"("image data"=w3437, "path to BMP file"=w3433) -> ()  [unwired: 1 in, 9 out]
              }
            }
          }
        }
        n2359 = node-c288(w3308) -> ()  [unwired: 1 out]
      }
      n2360 = node-c288(w3292) -> ()  [unwired: 1 out]
      n2361 = call "DMR_CloseDevice.vi"("driver handle IN"=w3297) -> ()  [unwired: 1 in, 4 out]
    }
    frame #4 {
      n2362 = call "DMR_Close.vi"() -> ()  [unwired: 1 out]
    }
  }
  n2363 = node-c288(i64 1 ("Period"), 1 ("Processor")) -> (w73:T23)  [unwired: 2 out]
  n2364 = timed-loop "Main data acquisition loop (get data, process data for display, and save data to disk)" {
    tunnel: w11 -> [w3761]
    tunnel: w10 -> [w3760]
    tunnel: [w3789] -> w80
    tunnel: [w3784] -> w79
    timing: w73 -> [_]
    timing-out: [_] -> w72
    tunnel: w47 -> [w3615]
    stop <- "Stop All" stop-if-true
    w3532 = "Initialize"
    # "T2 sum"
    # "T1 sum"
    # "Fluorescence data into FIFO for external control vi's\n(e.g., fluorescence triggering) - Duncan Nall"
    n2365 = node-c288() -> ()  [unwired: 2 out]
    n2366 = First Call?() -> (First Call?: T/F=w3567:bool)
    n2367 = Or(x="Reset", y=w3567) -> (x .or. y?=w3568:bool)
    n2368 = local read "Flushing P1"() -> (w3487:bool)
    n2369 = case "Reset data stream (manual reset or at begining of some rastering and imaging)" shown="True" w3568 {
      tunnel: w3761 -> [w4830 w4838]
      tunnel: w3760 -> [w4829 w4837]
      tunnel: [w4830 w4832] -> w3756
      tunnel: [w4829 w4831] -> w3755
      frame False {
      }
      frame True {
        w4835 = TRUE ("AI to FIFO")
        n2370 = local write "Overflow (data lost)"(FALSE ("Overflow (data lost)")) -> ()
        n2371 = call "reset FPGA DMA.vi"("error in"=w4837, "FPGA VI Reference In"=w4838) -> ("error out"=w4833:errorcluster, "FPGA VI Reference Out"=w4834:T20)
        n2372 = xnode "Read/Write Control"("FPGA VI Reference In"=w4834, "error in"=w4833, "AI to FIFO"=w4835, "APD to FIFO"=w4835) -> ("FPGA VI Reference Out"=w4832:T20, "error out"=w4831:errorcluster)
      }
    }
    n2373 = case shown="True" w3487 {
      frame False {
      }
      frame True {
        n2374 = local read "Flush rate (uL/m) P1"() -> (w3819:dbl)
        n2375 = local read "HP1 Flush Time (s)"() -> (w3828:dbl)
        n2376 = local read "DMA Update Period (s)"() -> (w3822:dbl)
        n2377 = Divide(x=w3819, y=60.0) -> (x/y=w3820:dbl)
        n2378 = Divide(x=w3828, y=w3822) -> (x/y=w3817:dbl)
        n2379 = feedback #4(0) -> (w3826:i32)
        n2380 = Increment(x=w3826) -> (x+1=w3816:i32)
        n2381 = Greater?(x=w3816, y=w3817) -> (0:w3825:bool)
        n2382 = Compound Arithmetic op=MULTIPLY(w3822, w3816, w3820) -> (→"P1 Flush Volume (uL)":dbl)
        n2383 = Divide(x=w3816, y=w3817) -> (x/y=→"P1 Flushing Bar":dbl)
        n2384 = case shown="True" w3825 {
          tunnel: w3816 -> [w3829 _]
          tunnel: [w3829 0] -> w3824
          frame False {
          }
          frame True {
            w3830 = FALSE ("Flushing P1")
            n2385 = local write "Inject Pump 1"(w3830) -> ()
            n2386 = local write "Flushing P1"(w3830) -> ()
            n2387 = property on="Clear Volume P1" class="Bool (strict)"("Val(Sgnl)"=TRUE ("Value (Signaling)")) -> ()  [unwired: 2 in, 2 out]
          }
        }
        n2388 = feedback-in #4(w3824) -> ()
      }
    }
    n2389 = Or(x="Start AOD Scan", y="Trap Raster Scan") -> (x .or. y?=w3712:bool)
    n2390 = case "Start AOM raster scan" shown="True" w3712 {
      tunnel: w3756 -> [w4680 w4690]
      tunnel: w3755 -> [w4679 w4689]
      tunnel: [w4680 w4683] -> w3754
      tunnel: [w4679 w4682] -> w3753
      frame False {
      }
      frame True {
        n2391 = case shown="True" "Restart DMA? (AOD)" {
          tunnel: [w4728 w4730] -> w4684
          tunnel: [w4727 w4729] -> w4685
          tunnel: w4690 -> [w4728 w4732]
          tunnel: w4689 -> [w4727 w4731]
          frame False {
          }
          frame True {
            n2392 = local write "Overflow (data lost)"(FALSE ("Overflow (data lost)")) -> ()
            n2393 = call "reset FPGA DMA.vi"("error in"=w4731, "FPGA VI Reference In"=w4732) -> ("error out"=w4729:errorcluster, "FPGA VI Reference Out"=w4730:T20)
          }
        }
        n2394 = local write "Trap Raster Scan"(FALSE ("Trap Raster Scan")) -> ()
        n2395 = case shown="True" "Move MCL Also?" {
          tunnel: w4685 -> [w4693 w4722]
          tunnel: w4684 -> [w4694 w4723]
          tunnel: [w4692 w4726] -> w4683
          tunnel: [w4691 w4725] -> w4682
          frame False {
            w4695 = TRUE ("AI to FIFO")
            n2396 = xnode "Read/Write Control"("FPGA VI Reference In"=w4694, "error in"=w4693, "AI to FIFO"=w4695, "APD to FIFO"=w4695, "Start scan"=w4695) -> ("FPGA VI Reference Out"=w4692:T20, "error out"=w4691:errorcluster)
          }
          frame True {
            w4719 = FALSE ("1D or 2D Scan?")
            w4724 = TRUE ("AI to FIFO")
            # "Count for MCL loop"
            # "N total cycles"
            # "N steps"
            # "V_int"
            n2397 = local read "Scan Range (nm)"() -> (w4701:dbl)
            n2398 = local read "Number of F/B Scans (AOD)"() -> (w4718:u16)
            n2399 = Sign(1:w4701) -> (0:w4700:dbl)
            n2400 = Compound Arithmetic op=MULTIPLY(w4701, "MCL Step Position Ratio", "MCL/AOM Scale Tweak") -> (w4705:dbl)
            n2401 = Negate(x=w4700) -> (-x=w4697:dbl)
            n2402 = Multiply(x=w4697, y="MCL Step Increment (V_int)") -> (x*y=w4699:dbl)
            n2403 = Divide(x=w4705, y="MCL X Cal (nm/V)") -> (x/y=w4711:dbl)
            n2404 = Multiply(x=32767.0 ("y"), y=w4711) -> (x*y=w4717:dbl)
            n2405 = local read "Total Counts (ticks)"() -> (w4702:u16)
            n2406 = local read "Cycles/step (AOD)"() -> (w4713:u64)
            n2407 = local read "Scan steps (AOD)"() -> (w4714:u64)
            n2408 = Divide(x=w4717, y=10.0) -> (x/y=w4710:dbl)
            n2409 = Divide(x=w4710, y="MCL Step Increment (V_int)") -> (x/y=w4708:dbl)
            n2410 = Absolute Value(x=w4708) -> (abs(x)=w4696:dbl)
            n2411 = Compound Arithmetic op=MULTIPLY(w4714, w4713, w4702) -> (w4709:u64)
            n2412 = local write "wait to reset values"(w4724) -> ()
            n2413 = local write "MCL Scanning"(w4724) -> ()
            n2414 = Divide(x=w4709, y=w4696) -> (x/y=w4706:dbl)
            "MCL Count" <- w4706
            n2415 = xnode "Read/Write Control"("FPGA VI Reference In"=w4723, "error in"=w4722, "Scan steps (MCL)"=w4696, "Number of scans (MCL)"=w4718, "Cycles per step (MCL)"=u64 1, "Scan freq.  increment (MCL)"=w4699, "1D or 2D Scan?"=w4719, "MCL Scan Axis"=w4719, "Cont. Scan (MCL)"=w4719, "MCL count"=w4706) -> ("FPGA VI Reference Out"=w4721:T20, "error out"=w4720:errorcluster)
            n2416 = xnode "Read/Write Control"("FPGA VI Reference In"=w4721, "error in"=w4720, "AI to FIFO"=w4724, "APD to FIFO"=w4724, "Start scan"=w4724, "Start scan (MCL)"=w4724) -> ("FPGA VI Reference Out"=w4726:T20, "error out"=w4725:errorcluster)
          }
        }
        "Raster Scanning..." <- TRUE ("Scanning...")
      }
    }
    n2417 = local read "Flushing P3"() -> (w3488:bool)
    n2418 = case "Keep track of when Harvard Pump 3 is done flushing" shown="True" w3488 {
      frame False {
      }
      frame True {
        n2419 = local read "Flush rate (uL/m) P3"() -> (w3836:dbl)
        n2420 = local read "DMA Update Period (s)"() -> (w3838:dbl)
        n2421 = local read "HP3 Flush Time (s)"() -> (w3845:dbl)
        n2422 = Divide(x=w3836, y=60.0) -> (x/y=w3834:dbl)
        n2423 = feedback #5(0) -> (w3843:i32)
        n2424 = Increment(x=w3843) -> (x+1=w3837:i32)
        n2425 = Divide(x=w3845, y=w3838) -> (x/y=w3839:dbl)
        n2426 = Greater?(x=w3837, y=w3839) -> (0:w3842:bool)
        n2427 = Compound Arithmetic op=MULTIPLY(w3838, w3837, w3834) -> (→"P3 Flush Volume (uL)":dbl)
        n2428 = case shown="True" w3842 {
          tunnel: w3837 -> [w3846 _]
          tunnel: [w3846 0] -> w3841
          frame False {
          }
          frame True {
            w3847 = FALSE ("Flushing P3")
            n2429 = local write "Inject Pump 3"(w3847) -> ()
            n2430 = local write "Flushing P3"(w3847) -> ()
            n2431 = property on="Clear Volume P3" class="Bool (strict)"("Val(Sgnl)"=TRUE ("Value (Signaling)")) -> ()  [unwired: 2 in, 2 out]
          }
        }
        n2432 = feedback-in #5(w3841) -> ()
        n2433 = Divide(x=w3837, y=w3839) -> (x/y=→"P3 Flushing Bar":dbl)
      }
    }
    n2434 = And(x="Save scans", y=w3712) -> (x .and. y?=w3752:bool)
    n2435 = Compound Arithmetic op=OR("Start MCL Scan", "Confocal Image", "Confocal Linescan") -> (w3710:bool)
    n2436 = And(x="Save Data (MCL)", y=w3710) -> (x .and. y?=w3751:bool)
    n2437 = case "Start MCL raster scan" shown="True" w3710 {
      tunnel: w3754 -> [w4292 w4308]
      tunnel: w3753 -> [w4291 w4307]
      tunnel: [w4292 w4303] -> w3614
      tunnel: [w4291 w4302] -> w3613
      tunnel: [FALSE w4301] -> w3737
      tunnel: "Start MCL Scan" -> [_ w4296]
      tunnel: "Confocal Image" -> [_ w4295]
      tunnel: "Confocal Linescan" -> [_ _]
      frame False {
      }
      frame True {
        w4301 = TRUE
        n2438 = case shown="True" "Restart DMA? (MCL)" {
          tunnel: [w4353 w4355] -> w4306
          tunnel: [w4352 w4354] -> w4305
          tunnel: w4308 -> [w4353 w4358]
          tunnel: w4307 -> [w4352 w4357]
          frame False {
          }
          frame True {
            n2439 = call "reset FPGA DMA.vi"("error in"=w4357, "FPGA VI Reference In"=w4358) -> ("error out"=w4354:errorcluster, "FPGA VI Reference Out"=w4355:T20)
            n2440 = local write "Overflow (data lost)"(FALSE ("Overflow (data lost)")) -> ()
          }
        }
        n2441 = case shown="False" w4296 {
          selector: w4296 -> [_ w4312]
          tunnel: w4295 -> [w4311 _]
          tunnel: [w4311 w4312] -> w4294
          frame False {
            n2442 = property on="2D or 1D Scan" class="Bool (strict)"("Val(Sgnl)"=w4311) -> ()  [unwired: 2 in, 2 out]
            n2443 = property on="Confocal Image" class="Bool (strict)"("Value"=FALSE ("Start Confocal Map")) -> ()  [unwired: 2 in, 2 out]
          }
          frame True {
          }
        }
        n2444 = local write "MCL Scanning"(w4301) -> ()
        n2445 = local read "AO1"() -> (w4298:dbl)
        n2446 = local read "AO2"() -> (w4297:dbl)
        n2447 = case shown="True" "Center Scan" {
          tunnel: w4306 -> [w4319 w4351]
          tunnel: w4305 -> [w4318 w4350]
          tunnel: [w4317 w4349] -> w4303
          tunnel: [w4316 w4348] -> w4302
          tunnel: [w4314 w4335] -> w4300
          tunnel: [w4313 w4334] -> w4299
          tunnel: w4298 -> [w4314 w4340]
          tunnel: w4297 -> [w4313 w4343]
          tunnel: w4294 -> [_ _]
          frame False {
            w4315 = TRUE ("AI to FIFO")
            n2448 = xnode "Read/Write Control"("FPGA VI Reference In"=w4319, "error in"=w4318, "AI to FIFO"=w4315, "APD to FIFO"=w4315, "Start scan (MCL)"=w4315) -> ("FPGA VI Reference Out"=w4317:T20, "error out"=w4316:errorcluster)